vi "pharmaBot_v0.019.vi"() -> ()   [LabVIEW 2015] (continued)
        n1090 = property on="Accept Button" class="Bool (strict)"("DisabledEnum"=T56."Enabled" ("Disabled")) -> ()  [unwired: 2 in, 2 out]
      }
      event "Cancel Calibration Button", "Redo Calibration Button": Mouse Up {
        n1091 = event-data() -> ()  [unwired: 1 in, 8 out]
        n1092 = local write "Calibration Protocol"(T7."Init" ("Calibration Protocol")) -> ()
        n1093 = property on="Accept Button" class="Bool (strict)"("DisabledEnum"=T56."Enabled" ("Disabled")) -> ()  [unwired: 2 in, 2 out]
        n1094 = local write "Stage zeroed?"(FALSE ("Stage zeroed")) -> ()
        n1095 = invoke on="Manip 3 Calibrated" class="Bool (strict)" method="Reinit To Default"() -> ()  [unwired: 3 in, 3 out]
        n1096 = invoke on="Manip 2 Calibrated" class="Bool (strict)" method="Reinit To Default"() -> ()  [unwired: 3 in, 3 out]
        n1097 = invoke on="Manip 1 Calibrated" class="Bool (strict)" method="Reinit To Default"() -> ()  [unwired: 3 in, 3 out]
        n1098 = invoke on="Manip 4 Calibrated" class="Bool (strict)" method="Reinit To Default"() -> ()  [unwired: 3 in, 3 out]
        n1099 = invoke on="Stage zeroed?" class="Bool (strict)" method="Reinit To Default"() -> ()  [unwired: 3 in, 3 out]
      }
      event "wash bath location", "set safe space", "location above baths", "cleaning bath location", "Zero Pipette 1": Mouse Up {
        n1100 = event-data() -> ()  [unwired: 1 in, 8 out]
        n1101 = property on="Accept Button" class="Bool (strict)"("DisabledEnum"=T56."Enabled" ("Disabled")) -> ()  [unwired: 2 in, 2 out]
      }
      event "Pipette is in Focus": Value Change {
        n1102 = event-data() -> ("NewVal"=w1408:bool)  [unwired: 1 in, 5 out]
        n1103 = case shown="True" w1408 {
          frame False {
          }
          frame True {
            n1104 = local read "Current Manipulator Position"() -> (→"Current Manip Focus Coords.":i32[])
            n1105 = local write "Pipette is in Focus?"(TRUE ("Pipette is in Focus?")) -> ()
          }
        }
      }
      event "Move Stage and Pipette Down": Value Change {
        n1106 = event-data() -> ("NewVal"=w1413:bool)  [unwired: 1 in, 5 out]
        n1107 = case shown="True" w1413 {
          tunnel: w1412 -> [_ w1427]
          tunnel: w1411 -> [_ w1426]
          frame False {
          }
          frame True {
            # "manip <z>"
            # "Shift stage by deltaZ"
            # "manip position <x,y>"
            # "calculate deltaZ, reset min on slider"
            # "stage position <x,y>"
            n1108 = local read "current stage pos (steps)"() -> (w1437:i32[])
            n1109 = local read "Next Stage and Pipette Z Location"() -> (w1439:dbl)
            n1110 = local read "Current Manipulator Position"() -> (w1433:i32[])
            n1111 = Index Array(array=w1437, index=2) -> (element=w1434:i32)
            n1112 = Array Subset(array=w1437, length=2) -> (w1430:i32[])  [unwired: 1 in]
            n1113 = Array Subset(array=w1433, length=2) -> (w1429:i32[])  [unwired: 1 in]
            n1114 = Round To Nearest(number=w1439) -> (nearest integer value=w1428:dbl)
            n1115 = flat-sequence {
              tunnel: w1427 -> [w1445]
              tunnel: w1426 -> [w1440]
              tunnel: w1425 -> [w1443]
              tunnel: [w1441] -> w1424
              tunnel: [w1440] -> w1423
              tunnel: w1424 -> [_]
              tunnel: w1423 -> [w1452]
              tunnel: w1422 -> [w1448]
              tunnel: [w1446] -> _
              frame #0 {
                # "move the pipette..."
                n1116 = local read "Calibrate:"() -> (w1444:T8)
                n1117 = call "move manipulator abs xyz.vi"("blocking?"=TRUE, "which manipulator"=w1444, "transform cluster + actuator"=w1440, "positions"=w1445, "location (steps)"=w1443) -> ("error out"=w1441:errorcluster)  [unwired: 6 in]
              }
              frame #1 {
                # "then the stage..."
                n1118 = Unbundle By Name(w1452) -> ("s"=w1451:refnum<vi>)
                n1119 = property class="Clust (strict)"(reference=w1451) -> ("Value"=w1450:T25)  [unwired: 1 in, 2 out]
                n1120 = Unbundle By Name(w1450) -> ("actuator"=w1449:T26)
                n1121 = call "moveTo_abs_XYZ.vi"("blocking?"=TRUE, "XYZ location (steps)"=w1448, "Actuator cluster in"=w1449) -> ("error out"=w1446:errorcluster)  [unwired: 7 in, 1 out]
              }
            }
            n1122 = Subtract(x=w1434, y=w1428) -> (x-y=w1418:dbl)
            n1123 = Index Array(array=w1433, index=2) -> (element=w1432:i32)
            n1124 = Divide(x=w1418, y=7.53) -> (x/y=w1416:dbl)
            n1125 = Subtract(x=w1432, y=w1416) -> (x-y=w1415:dbl)
            n1126 = Subtract(x=w1434, y=w1418) -> (x-y=w1421:dbl)
            n1127 = Negate(x=w1415) -> (-x=w1414:dbl)
            n1128 = Multiply(x=w1421, y=1.0) -> (x*y=w1419:dbl)
            n1129 = Build Array (concatenate)(w1429, w1414) -> (w1425:dbl[])
            "next manip position" <- w1425
            n1130 = Build Array (concatenate)(w1430, w1419) -> (w1422:dbl[])
            "next stage position" <- w1422
          }
        }
      }
      event "Stage Shift (steps)": Value Change {
        n1131 = event-data() -> ("NewVal"=w1453:dbl)  [unwired: 1 in, 5 out]
        n1132 = property on="Next Stage and Pipette Z Location" class="Slide (strict)"("Scale.Maximum"=w1453) -> ()  [unwired: 2 in, 2 out]
      }
      event "Accept Button": Mouse Up {
        n1133 = event-data() -> ()  [unwired: 1 in, 8 out]
        n1134 = property on="Accept Button" class="Bool (strict)"("DisabledEnum"=T56."Disabled and Grayed Out" ("Disabled")) -> ()  [unwired: 2 in, 2 out]
      }
      event "Seek Backwards Calibration Button": Mouse Up {
        n1135 = event-data() -> ()  [unwired: 1 in, 8 out]
        n1136 = local read "Calibration Protocol"() -> (w1457:T7)
        n1137 = Decrement(x=w1457) -> (x-1=w1456:T7)
        n1138 = local write "Calibration Protocol"(w1456) -> ()
        n1139 = property on="Accept Button" class="Bool (strict)"("DisabledEnum"=T56."Disabled and Grayed Out" ("Disabled")) -> ()  [unwired: 2 in, 2 out]
      }
    }
  }
  n1140 = Merge Errors(w395, w396) -> (w397:errorcluster)
  n1141 = case shown="True" w253 {
    tunnel: w467 -> [_ w1466]
    tunnel: w245 -> [_ w1465]
    tunnel: w520 -> [_ w1464]
    tunnel: w518 -> [_ w1463]
    tunnel: w249 -> [_ w1462]
    tunnel: T8."manipulator 2" ("which manipulator") -> [_ w1461]
    tunnel: w281 -> [_ w1460]
    tunnel: w278 -> [_ _]
    frame False {
    }
    frame True {
      n1142 = Current VI's Path() -> (path=w1459:path)
      n1143 = control-ref of="allMainVIcontrols"() -> (w1458:refnum<vi>)
      n1144 = call "multipatch_states_V0.030_dualWCedits.vi"("common cluster"=w1465, "images"=w1466, "allMainVIcontrols"=w1458, "which manipulator"=w1461, "individual controls in"=w1462, "state in"=w1463, "cam size"=w1460, "time in"=w1464, "mainVIpath"=w1459) -> ()  [unwired: 6 in, 1 out]
    }
  }
  n1145 = local write "pipette 2 template"(w267) -> ()
  n1146 = local read "Adjust exposure (ms)"() -> (w275:dbl)
  n1147 = Not(x=w703) -> (.not. x?=→"initialized":bool)
  n1148 = case shown="True" w251 {
    tunnel: w471 -> [_ w1475]
    tunnel: w245 -> [_ w1474]
    tunnel: w520 -> [_ w1473]
    tunnel: w518 -> [_ w1472]
    tunnel: w246 -> [_ w1471]
    tunnel: T8."manipulator 1" ("which manipulator") -> [_ w1470]
    tunnel: w281 -> [_ w1469]
    tunnel: w278 -> [_ _]
    frame False {
    }
    frame True {
      n1149 = Current VI's Path() -> (path=w1468:path)
      n1150 = control-ref of="allMainVIcontrols"() -> (w1467:refnum<vi>)
      n1151 = call "multipatch_states_V0.030_dualWCedits.vi"("common cluster"=w1474, "images"=w1475, "allMainVIcontrols"=w1467, "which manipulator"=w1470, "individual controls in"=w1471, "state in"=w1472, "cam size"=w1469, "time in"=w1473, "mainVIpath"=w1468) -> ()  [unwired: 6 in, 1 out]
    }
  }
  n1152 = while {
    tunnel: w378 -> [w1502]
    tunnel: w336 -> [w1501]
    tunnel: w338 -> [w1495]
    stop <- w1507 stop-if-true
    n1153 = local read "measured manip 1 zero (steps)"() -> (w1497:i32[])
    n1154 = local read "measured stage zero (steps)"() -> (w1496:i32[])
    n1155 = call "get_XYZ.vi"("Actuator cluster in"=w1495) -> ("X pos (steps)"=w1494:i32, "Y pos (steps)"=w1493:i32, "Z pos (steps)"=w1492:i32)  [unwired: 10 in, 2 out]
    n1156 = call "get_XYZ.vi"("Actuator cluster in"=w1502) -> ("X pos (steps)"=w1506:i32, "Y pos (steps)"=w1505:i32, "Z pos (steps)"=w1500:i32)  [unwired: 10 in, 2 out]
    n1157 = call "get_XYZ.vi"("Actuator cluster in"=w1501) -> ("X pos (steps)"=w1504:i32, "Y pos (steps)"=w1503:i32, "Z pos (steps)"=w1499:i32)  [unwired: 10 in, 2 out]
    n1158 = Build Array(w1506, w1505, w1500) -> (w1498:i32[])
    n1159 = Build Array(w1504, w1503, w1499) -> (w1486:i32[])
    n1160 = Build Array(w1494, w1493, w1492) -> (w1491:i32[])
    n1161 = Subtract(x=w1498, y=w1497) -> (x-y=w1477:i32[])
    n1162 = Subtract(x=w1486, y=w1496) -> (x-y=w1478:i32[])
    n1163 = local write "current manip 2 pos (steps)"(w1491) -> ()
    n1164 = local write "measured stage difference (steps)"(w1478) -> ()
    n1165 = local write "current manip 1 pos (steps)"(w1498) -> ()
    n1166 = local write "current stage pos (steps)"(w1486) -> ()
    n1167 = call-poly <vilib>:"nrm2 - Vector 2-Norm.vi"("x"=w1477) -> ("dnrm2"=w1476:dbl)  [unwired: 9 in, 1 out]
    n1168 = call-poly <vilib>:"nrm2 - Vector 2-Norm.vi"("x"=w1478) -> ("dnrm2"=w1479:dbl)  [unwired: 9 in, 1 out]
    n1169 = local write "stage distance (steps)"(w1479) -> ()
    n1170 = local write "measured manip 1 difference (steps)"(w1477) -> ()
    n1171 = local read "stop always"() -> (w1507:bool)
    n1172 = local write "manip distance (steps)"(w1476) -> ()
    n1173 = Index Array(array=w1486, index=2) -> (element=w1484:i32)
    n1174 = Array Subset(array=w1486, length=2) -> (w1483:i32[])  [unwired: 1 in]
    n1175 = Wait (ms)(milliseconds to wait=u32 100) -> ()  [unwired: 1 out]
    n1176 = Divide(x=w1484, y=-75.3) -> (x/y=w1488:dbl)
    n1177 = Divide(x=w1483, y=10 ("Z pos (steps)")) -> (x/y=w1481:dbl[])
    n1178 = Insert Into Array(array=w1481, index=2, new element=w1488) -> (w1480:dbl[])
    n1179 = local write "current stage pos [um]"(w1480) -> ()
  }
  n1180 = And(x=w251, y=w253) -> (x .and. y?=w411:bool)
  n1181 = Bundle By Name(cluster=T38 {"camera type"=enum."optiMOS", "cam handle"=16842752, "data handle"=0, "cam size"=[]} ("cam info in"), "camera type"=w277) -> (w662:T38)
  n1182 = call "init_cam_topLvl_v02.vi"("exposure (ms)"=w275, "orig image"=w276, "cam info in"=w662) -> ("error out"=w280:errorcluster, "cam info out"=w273:T38)  [unwired: 7 in]
  n1183 = Unbundle By Name(w273) -> ("cam size"=w328:i32[])
  n1184 = call "IMAQ Create"("Border Size"=0, "Image Name"="correctionMask", "Image Type"=w332, "error in (no error)"=w333) -> ("New Image"=w329:T10, "error out"=w330:errorcluster)  [unwired: 1 in]
  n1185 = call <vilib>:"Set Plots.vi"("3D graph"=w271, "# of plots(1)"=7) -> ("3D graph out"=w666:refnum<k7>, "error out"=w665:errorcluster)  [unwired: 12 in]
  n1186 = local write "Select cells based on proximity (multi patch)"(w411) -> ()
  n1187 = local read "cell diameter (px)"() -> (w274:i32)
  n1188 = local write "cam info out"(w273) -> ()
  n1189 = Index Array(array=w328) -> (element #1=w327:i32, element #2=w326:i32)  [unwired: 2 in]
  n1190 = call "condition3dplot_v02.vi"("error in"=w665, "3d graph"=w666) -> ("3d graph out"=w664:refnum<k7>)  [unwired: 8 in, 1 out]
  n1191 = property class="CWGraph3D"(reference=w271) -> ("Axes"=w635:refnum<k7>)  [unwired: 1 in, 2 out]
  n1192 = call "IMAQ SetImageSize"("error in (no error)"=w330, "Y Resolution"=w326, "X Resolution"=w327, "Image"=w329) -> ("error out"=w325:errorcluster, "Image Out"=w324:T10)  [unwired: 1 in]
  n1193 = Select(t=scope_motion."slow_dualPatch" ("motion"), s=w411, f=scope_motion."slow_dualPatch" ("motion")) -> (s? t:f=w248:T19)
  n1194 = flat-sequence {
    tunnel: [w1513] -> w637
    tunnel: [w1512] -> w636
    tunnel: w273 -> [w1511]
    tunnel: w280 -> [w1510]
    tunnel: [w1510] -> w279
    frame #0 {
      n1195 = Unbundle By Name(w1511) -> ("cam size"=w1509:i32[])
      n1196 = Index Array(array=w1509) -> (element #1=w1513:i32, element #2=w1512:i32)  [unwired: 2 in]
      n1197 = local write "cam size"(w1509) -> ()
      n1198 = property on="camera" class="XYGraph (strict)"("XScale.Maximum"=w1513, "YScale.Maximum"=w1512) -> ()  [unwired: 2 in, 2 out]
    }
  }
  n1199 = call "init_camCorrection.vi"("error in"=w325, "orig image"=w324, "cam info in"=w273) -> ("error out"=w282:errorcluster, "orig image out"=w323:T10)  [unwired: 7 in]
  n1200 = local write "pipette motion"(w248) -> ()
  n1201 = To Variant(anything=1) -> (Variant=w644:variant)
  n1202 = To Variant(anything=2) -> (Variant=w642:variant)
  n1203 = local read "Valve2 Connected"() -> (w283:bool)
  n1204 = invoke class="CWAxes3D" method="Item"(reference=w635, "Item"=w642) -> ("Item"=w640:refnum<k7>)  [unwired: 2 in, 3 out]
  n1205 = invoke class="CWAxes3D" method="Item"(reference=w635, "Item"=w644) -> ("Item"=w643:refnum<k7>)  [unwired: 2 in, 3 out]
  n1206 = local read "P1 state"() -> (w356:T11)
  n1207 = while {
    tunnel: w276 -> [w1547]
    tunnel: [w1521] -> w681
    tunnel: [w1523] -> w680
    tunnel: [w1554] -> w677
    tunnel: [w1553] -> w676
    tunnel: w274 -> [w1555]
    tunnel: w366 -> [w1520]
    tunnel: w273 -> [w1548]
    tunnel: w280 -> [w1546]
    tunnel: [w1525] -> w660
    shift-right: [w1516] -> _
    shift-left: sgl[] [] ("Distances") -> [w1537]
    tunnel: w275 -> [w1529]
    tunnel: w282 -> [_]
    tunnel: w323 -> [w1519]
    stop <- w1559 stop-if-true
    w1541 = i32[] [2] items=["No Event"=0, "Click Event"=1, "Draw Event"=2, "Size Event"=4, "Scroll Event"=5, "Double Click Event"=8] ("Which Events")
    # "draws circle where it found tip\nduring auto pipette calibration"
    # "if cell tracker is ON\nplot outline, centroid, pipette position"
    n1208 = local read "Vision Fix"() -> (w1526:bool)
    n1209 = call "grab_image_topLvl_v02.vi"("error in"=w1546, "orig image"=w1547, "cam info in"=w1548) -> ("error out"=w1522:errorcluster, "orig image out"=w1524:T10, "cam info out"=w1525:T38)  [unwired: 6 in]
    n1210 = Multiply(x=w1529, y=1.1) -> (x*y=w1527:dbl)
    n1211 = case shown="True" w1526 {
      tunnel: w1524 -> [w1561 w1563]
      tunnel: [w1561 w1567] -> w1523
      tunnel: w1522 -> [w1560 w1565]
      tunnel: [w1560 w1564] -> w1521
      tunnel: w1520 -> [_ w1566]
      tunnel: w1519 -> [_ w1562]
      frame False {
      }
      frame True {
        n1212 = call "IMAQ Multiply"("Image Src A"=w1563, "Image Dst"=w1566, "Image Src B"=w1562, "error in (no error)"=w1565) -> ("Image Dst Out"=w1567:T10, "error out"=w1564:errorcluster)  [unwired: 3 in]
      }
    }
    n1213 = Wait (ms)(milliseconds to wait=w1527) -> ()  [unwired: 1 out]
    n1214 = call "IMAQ Copy"("error in (no error)"=w1521, "Image Dst"=w1520, "Image Src"=w1523) -> ("error out"=w1545:errorcluster, "Image Dst Out"=w1544:T10)  [unwired: 3 in]
    n1215 = local read "crosshair?"() -> (w1517:bool)
    n1216 = case shown="True" w1517 {
      tunnel: [w1608 w1612] -> w1557
      tunnel: [w1607 w1611] -> w1556
      tunnel: w1544 -> [w1608 w1610]
      tunnel: w1545 -> [w1607 w1609]
      frame False {
      }
      frame True {
        n1217 = call "overlayCrosshairs.vi"("error in"=w1609, "Image in"=w1610) -> ("error out"=w1611:errorcluster, "Image out"=w1612:T10)  [unwired: 8 in]
      }
    }
    n1218 = local read "current cell locations (px)"() -> (w1558:dbl[][])
    n1219 = invoke on="Slice view" class="ImageControl" method="Get Last Event"("Which Events"=w1541) -> ("Tool"=w1536:i32, "Coordinates"=w1540:i32[])  [unwired: 7 in, 6 out]
    n1220 = call "drawCells.vi"("error in"=w1556, "diameter (px)"=w1555, "current cell locations (px)"=w1558, "Image in"=w1557) -> ("error out"=w1539:errorcluster, "Image out"=w1542:T10)  [unwired: 6 in]
    n1221 = case shown="3" w1536 {
      tunnel: w1540 -> [_ w1574]
      tunnel: w1539 -> [w1569 w1573]
      tunnel: [w1569 w1572] -> w1538
      tunnel: [w1568 w1570] -> w1516
      tunnel: w1537 -> [w1568 _]
      frame 0, Default {
      }
      frame 3 {
        w1571 = cluster{"X":sgl, "Y":sgl} {"X"=0.0, "Y"=0.0}
        # "Line tool"
        # "IMAQ Point Distances"
        n1222 = Index Array(array=w1574, index #1=0 ("index"), index #2=1 ("index"), index #3=2 ("index"), index #4=3 ("index")) -> (element #1=w1579:i32, element #2=w1580:i32, element #3=w1581:i32, element #4=w1582:i32)
        n1223 = Bundle(cluster=w1571, "X"=w1581, "Y"=w1582) -> (w1583:cluster{"X":sgl, "Y":sgl})
        n1224 = Bundle(cluster=w1571, "X"=w1579, "Y"=w1580) -> (w1584:cluster{"X":sgl, "Y":sgl})
        n1225 = Build Array(w1583, w1584) -> (w1585:cluster{"X":sgl, "Y":sgl}[])
        n1226 = call "IMAQ Point Distances"("Points"=w1585, "error in (no error)"=w1573) -> ("Distances"=w1570:sgl[], "error out"=w1572:errorcluster)  [unwired: 3 in]
      }
    }
    n1227 = local read "tracking"() -> (w1543:bool)
    n1228 = case shown="False" w1543 {
      tunnel: w1542 -> [w1587 w1605]
      tunnel: w1538 -> [w1586 w1604]
      tunnel: [w1586 w1588] -> w1534
      tunnel: [w1587 w1589] -> w1535
      frame False {
      }
      frame True {
        n1229 = local read "cell mask ROI"() -> (w1606:T28)
        n1230 = local read "centroid_px"() -> (w1598:dbl[])
        n1231 = call "IMAQ Overlay ROI"("error in (no error)"=w1604, "ROI Descriptor"=w1606, "Image"=w1605) -> ("error out"=w1599:errorcluster, "Image Out"=w1600:T10)  [unwired: 7 in]
        n1232 = To Long Integer(number=w1598) -> (32bit integer=w1597:i32[])
        n1233 = call "boundingBoxCoords.vi"("side length (px)"=20, "center (x,y)"=w1597) -> ("bounding box"=w1601:T59)  [unwired: 8 in, 1 out]
        n1234 = local read "pipette_px_onscreen"() -> (w1592:dbl[])
        n1235 = call "IMAQ Overlay Oval"("Color"=u32 6618880, "error in (no error)"=w1599, "Bounding Rectangle"=w1601, "Image"=w1600) -> ("error out"=w1590:errorcluster, "Image Out"=w1591:T10)  [unwired: 6 in]
        n1236 = To Long Integer(number=w1592) -> (32bit integer=w1596:i32[])
        n1237 = call "boundingBoxCoords.vi"("side length (px)"=10, "center (x,y)"=w1596) -> ("bounding box"=w1595:T59)  [unwired: 8 in, 1 out]
        n1238 = call "IMAQ Overlay Oval"("Color"=u32 9567230, "error in (no error)"=w1590, "Bounding Rectangle"=w1595, "Image"=w1591) -> ("error out"=w1588:errorcluster, "Image Out"=w1589:T10)  [unwired: 6 in]
      }
    }
    n1239 = local write "Distances"(w1516) -> ()
    n1240 = local read "Range"() -> (w1515:cluster{"Minimum":sgl, "Maximum":sgl})
    n1241 = call "IMAQ MathLookup"("Range"=w1515, "Operator"=T58."Linear", "error in (no error)"=w1534, "Image Src"=w1535) -> ("error out"=w1532:errorcluster, "Image Dst Out"=w1518:T10)  [unwired: 6 in]
    n1242 = call "IMAQ Histograph"("Interval Range"=w1515, "Image"=w1518) -> ("Histogram Graph"=w1514:T21)  [unwired: 6 in, 3 out]
    n1243 = local read "screen tip location (px)"() -> (w1549:i32[])
    n1244 = local write "Waveform Graph"(w1514) -> ()
    n1245 = local write "Slice view"(w1518) -> ()
    n1246 = local read "stop always"() -> (w1559:bool)
    n1247 = call "_Adjust Dynamic_simple.vi"("error in (no error)"=w1532, "Image Src"=w1518) -> ("error out"=w1531:errorcluster, "Image Out"=w1530:T10)  [unwired: 8 in]
    n1248 = call "boundingBoxCoords.vi"("side length (px)"=20, "center (x,y)"=w1549) -> ("bounding box"=w1551:T59)  [unwired: 8 in, 1 out]
    n1249 = call "IMAQ Overlay Oval"("Color"=u32 16711680, "error in (no error)"=w1531, "Bounding Rectangle"=w1551, "Image"=w1530) -> ("error out"=w1553:errorcluster, "Image Out"=w1554:T10)  [unwired: 6 in]
  }
  n1250 = local read "P1 state"() -> (w353:T11)
  n1251 = Not Equal?(x=w353, y=user_message_v6."Setting defaults..." ("P1 state")) -> (x != y?=w357:bool)
  n1252 = Not Equal?(x=w356, y=user_message_v6."Initializing..." ("P1 state")) -> (x != y?=w358:bool)
  n1253 = Or(x=w357, y=w358) -> (x .or. y?=w285:bool)
  n1254 = Select(t=w285, s=w283, f=w283) -> (s? t:f=w284:bool)
  n1255 = control-ref of="Command pressure (mBar) 1"() -> (w670:refnum<vi>)
  n1256 = while {
    tunnel: w270 -> [w1623]
    tunnel: w272 -> [w1622]
    tunnel: w664 -> [w1619]
    tunnel: [w1619] -> w663
    stop <- w1621 stop-if-true
    n1257 = local read "park plane z (px)"() -> (w1618:dbl)
    n1258 = local read "cells (image px)"() -> (w1620:dbl[][])
    n1259 = call "cam5_3dTest.vi"("park plane z (px)"=w1618, "3d graph"=w1619, "transform cluster + actuator"=w1622, "positions"=w1623, "cells (image px locations)"=w1620) -> ("current stage location (px)"=w1613:dbl[], "current pipette locations (px)"=w1614:dbl[][], "current cell locations (px)"=w1615:dbl[][], "currentState out"=w1616:T33, "current park plane z (px)"=w1617:dbl)  [unwired: 2 in]
    n1260 = local write "current park plane z (px)"(w1617) -> ()
    n1261 = local write "camera"(w1616) -> ()
    n1262 = local write "current cell locations (px)"(w1615) -> ()
    n1263 = local write "current pipette locations (px)"(w1614) -> ()
    n1264 = local write "current stage location (px)"(w1613) -> ()
    n1265 = local read "stop always"() -> (w1621:bool)
    n1266 = Wait (ms)(milliseconds to wait=u32 100) -> ()  [unwired: 1 out]
  }
  n1267 = call "Time Delay2"("Delay Time (s)"=2.0) -> ("error out"=w701:errorcluster)  [unwired: 10 in]
  n1268 = To Variant(anything=w636) -> (Variant=w638:variant)
  n1269 = To Variant(anything=w637) -> (Variant=w639:variant)
  n1270 = property class="CWAxis3D"(reference=w640, "Maximum"=w638) -> ()  [unwired: 1 in, 2 out]
  n1271 = property class="CWAxis3D"(reference=w643, "Maximum"=w639) -> ()  [unwired: 1 in, 2 out]
  n1272 = local read "demo daq?"() -> (w247:bool)
  n1273 = control-ref of="Command pressure (mBar) 2"() -> (w482:refnum<vi>)
  n1274 = while {
    tunnel: w696 -> [w1649]
    tunnel: w266 -> [w1648]
    tunnel: w627 -> [w1647]
    tunnel: w270 -> [w1646]
    tunnel: w272 -> [w1645]
    tunnel: w672 -> [w1644]
    tunnel: w322 -> [w1643]
    tunnel: w670 -> [w1642]
    tunnel: w265 -> [w1641]
    tunnel: w621 -> [w1640]
    tunnel: w482 -> [w1639]
    tunnel: w267 -> [w1638]
    tunnel: w464 -> [w1637]
    tunnel: w269 -> [w1636]
    tunnel: w456 -> [w1635]
    tunnel: w432 -> [w1634]
    tunnel: w431 -> [w1633]
    tunnel: w394 -> [w1632]
    tunnel: w398 -> [w1631]
    tunnel: [w1630] -> w401
    tunnel: [w1629] -> w400
    tunnel: w366 -> [w1628]
    tunnel: w337 -> [w1627]
    tunnel: w246 -> [w1626]
    tunnel: w245 -> [w1625]
    stop <- w1650 stop-if-true
    n1275 = event shown="[29] \"MZ Dn\", \"MZ Up\", \"MX Up\", \"MX Dn\", \"MY Dn\", \"MY Up\", \"SZ Dn\", \"SZ Up\", \"SX Up\", \"SX Dn\", \"SY Dn\", \"SY Up\": Value Change" {
      selector: _ -> [_ _ _ _ _ _ _ _ _ _ _ _ _ _ _ _ _ _ _ _ _ _ _ _ _ _ _ _ _ _ _ _ _ _ _ _ _ _ _ _ _]
      dyn-events: _ -> [_ _ _ _ _ _ _ _ _ _ _ _ _ _ _ _ _ _ _ _ _ _ _ _ _ _ _ _ _ _ _ _ _ _ _ _ _ _ _ _ _]
      timeout: _ -> [_ _ _ _ _ _ _ _ _ _ _ _ _ _ _ _ _ _ _ _ _ _ _ _ _ _ _ _ _ _ _ _ _ _ _ _ _ _ _ _ _]
      tunnel: [w1653 FALSE ("stop events") TRUE ("stop events") FALSE ("stop events") FALSE ("stop events") TRUE ("stop events") FALSE ("stop events") FALSE ("stop events") FALSE ("stop events") FALSE ("stop events") _ FALSE ("stop events") FALSE ("stop events") FALSE ("stop events") FALSE ("stop events") FALSE ("stop events") FALSE ("stop events") FALSE ("stop events") FALSE ("stop events") FALSE ("stop events") FALSE ("stop events") FALSE ("stop events") FALSE ("stop events") FALSE ("stop events") FALSE ("stop events") FALSE ("stop events") FALSE ("stop events") FALSE ("stop events") FALSE ("stop events") FALSE ("stop events") FALSE ("stop events") FALSE ("stop events") FALSE ("stop events") FALSE ("stop events") _ _ FALSE ("stop events") FALSE ("stop events") FALSE ("stop events") FALSE ("stop events") FALSE ("stop events")] -> w1650
      tunnel: w1649 -> [_ _ _ _ _ _ _ _ _ _ _ _ _ _ _ _ _ _ _ _ _ _ w2190 w2219 _ _ _ _ _ _ _ _ w2703 _ _ _ _ _ _ _ _]
      tunnel: w1648 -> [_ _ _ _ _ _ w1723 _ _ _ _ _ _ _ _ _ _ _ _ _ _ _ _ _ _ _ _ _ _ _ _ _ _ _ _ _ _ _ _ _ _]
      tunnel: w1647 -> [_ _ _ _ _ _ w1727 _ _ _ _ _ _ _ _ _ _ _ _ _ _ _ _ _ _ _ _ _ _ _ _ _ _ _ _ _ _ _ _ _ _]
      tunnel: w1646 -> [_ _ w1661 _ _ w1695 w1726 _ _ w1915 _ _ _ _ _ _ _ _ _ _ _ w2170 w2192 w2221 w2246 w2275 _ w2341 w2380 w2416 w2642 w2670 _ _ _ _ _ _ _ _ w2866]
      tunnel: w1645 -> [_ _ w1662 _ _ w1696 w1725 w1895 _ w1914 _ _ _ _ _ w1986 w2022 w2092 w2112 w2132 w2147 w2169 w2193 w2222 w2249 w2278 w2308 w2342 w2381 w2417 w2643 w2669 _ _ _ _ _ _ _ _ w2865]
      tunnel: w1644 -> [_ _ _ _ _ _ _ _ _ _ _ _ _ w1951 _ _ _ _ _ _ _ _ _ _ _ _ _ _ _ _ _ _ _ _ _ _ _ _ _ _ _]
      tunnel: w1643 -> [_ _ w1664 w1687 w1691 w1698 _ _ _ _ _ _ _ _ _ _ _ _ _ _ _ _ _ _ _ _ _ _ _ _ _ _ _ _ _ _ _ _ _ _ _]
      tunnel: w1642 -> [_ _ w1663 w1686 _ w1697 _ _ _ _ _ _ _ _ _ _ _ _ _ _ _ _ _ _ _ _ _ _ _ _ _ _ _ _ _ _ _ _ _ _ _]
      tunnel: w1641 -> [_ _ _ _ _ _ w1724 _ _ _ _ _ _ _ _ _ _ _ _ _ _ _ _ _ _ _ _ _ _ _ _ _ _ _ _ _ _ _ _ _ _]
      tunnel: w1640 -> [_ _ _ _ _ _ w1722 _ _ _ _ _ _ _ _ _ _ _ _ _ _ _ _ _ _ _ _ _ _ _ _ _ _ _ _ _ _ _ _ _ _]
      tunnel: w1639 -> [_ _ _ _ w1690 w1694 _ _ _ _ _ _ _ _ _ _ _ _ _ _ _ _ _ _ _ _ _ _ _ _ _ _ _ _ _ _ _ _ _ _ _]
      tunnel: w1638 -> [_ _ _ _ _ _ w1721 _ _ _ _ _ _ _ _ _ _ _ _ _ _ _ _ _ _ _ _ _ _ _ _ _ _ _ _ _ _ _ _ _ _]
      tunnel: w1637 -> [_ _ _ _ _ _ w1720 _ _ _ _ _ _ _ _ _ _ _ _ _ _ _ _ _ _ _ _ _ _ _ _ _ _ _ _ _ _ _ _ _ _]
      tunnel: w1636 -> [_ _ _ _ _ _ w1719 _ _ _ _ _ _ _ _ _ _ _ _ _ _ _ _ _ _ _ _ _ _ _ _ _ _ _ _ _ _ _ _ _ _]
      tunnel: w1635 -> [_ _ _ _ _ _ w1718 _ _ _ _ _ _ _ _ _ _ _ _ _ _ _ _ _ _ _ _ _ _ _ _ _ _ _ _ _ _ _ _ _ _]
      tunnel: w1634 -> [_ _ _ _ _ _ w1716 _ _ _ _ _ _ _ _ _ _ _ _ _ _ _ _ _ _ _ _ _ _ _ _ _ _ _ _ _ _ _ _ _ _]
      tunnel: w1633 -> [_ _ _ _ _ _ w1715 _ _ _ _ _ _ _ _ _ _ _ _ _ _ _ _ _ _ _ _ _ _ _ _ _ _ _ _ _ _ _ _ _ _]
      tunnel: w1632 -> [w1655 _ _ _ _ _ _ _ _ _ _ _ _ _ _ _ _ _ _ _ _ _ _ _ _ _ _ _ _ _ _ _ _ _ _ _ _ _ _ _ _]
      tunnel: w1631 -> [w1654 w1658 _ _ _ _ _ _ _ _ _ _ _ _ _ _ _ _ _ _ _ _ _ _ _ _ _ _ _ _ _ _ _ _ _ _ _ _ _ _ _]
      tunnel: [w1652 _ _ _ _ _ _ _ _ _ _ _ _ _ _ _ _ _ _ _ _ _ _ _ _ _ _ _ _ _ _ _ _ _ _ _ _ _ _ _ _] -> w1630
      tunnel: [w1651 w1658 _ _ _ _ _ _ _ _ _ _ _ _ _ _ _ _ _ _ _ _ _ _ _ _ _ _ _ _ _ _ _ _ _ _ _ _ _ _ _] -> w1629
      tunnel: w1628 -> [_ _ _ _ _ _ w1714 w1896 _ w1913 _ _ _ _ _ _ w2021 _ _ _ _ _ _ _ _ _ _ _ _ _ _ _ _ _ _ _ _ _ _ _ _]
      tunnel: w1627 -> [_ _ _ _ _ _ _ _ _ _ _ _ _ _ _ _ _ _ _ _ _ _ w2191 w2220 w2248 w2277 _ _ _ _ _ _ _ _ _ _ _ _ _ _ _]
      tunnel: w1626 -> [_ _ _ _ _ _ _ _ _ _ _ _ _ _ _ _ _ _ _ _ _ _ w2189 w2218 w2247 w2276 _ _ _ _ _ _ _ _ _ _ _ _ _ _ _]
      tunnel: w1625 -> [_ _ _ _ _ _ _ _ _ _ _ _ _ _ _ _ _ _ _ _ _ _ w2188 w2217 _ _ _ _ _ _ _ _ _ _ _ _ _ _ _ _ _]
      event "stop": Value Change {
        w1653 = TRUE ("stop events")
        n1276 = event-data() -> ()  [unwired: 1 in, 5 out]
        n1277 = Send Notification(notification=w1653, notifier=w1655, error in (no error)=w1654) -> (notifier out=w1652:refnum<notifier>, error out=w1651:errorcluster)
        "stop always" <- TRUE ("stop always")
      }
      event Timeout {
        n1278 = event-data() -> ()  [unwired: 1 in, 3 out]
        n1279 = Wait (ms)(milliseconds to wait=u32 50) -> ()  [unwired: 1 out]
      }
      event "pipette 1 broken - abort!": Value Change {
        n1280 = event-data() -> ("NewVal"=w1665:bool)  [unwired: 1 in, 5 out]
        n1281 = case shown="True" w1665 {
          tunnel: w1664 -> [_ w1681]
          tunnel: w1663 -> [_ w1680]
          tunnel: w1662 -> [_ w1670]
          tunnel: w1661 -> [_ w1676]
          frame False {
          }
          frame True {
            w1675 = T8."manipulator 1" ("which manipulator")
            n1282 = Unbundle By Name(w1670) -> ("manip 1"=w1669:refnum<vi>)
            n1283 = property class="Clust (strict)"(reference=w1669) -> (error out=w1668:errorcluster, "Value"=w1667:T25)  [unwired: 1 in, 1 out]
            n1284 = call "switchPressure_topLvl.vi"("which manipulator"=w1675, "Slide Refnum"=w1680, "error in"=w1668, "pressure setting"=arduino_pressure_setting."Atmospheric Pressure", "Pressure box control in"=w1681) -> ("error out"=w1671:errorcluster)  [unwired: 5 in, 1 out]
            n1285 = Unbundle By Name(w1667) -> ("actuator.Actuator COM"=w1672:refnum<visa-resource-name>)
            n1286 = call "sc_adjustMotion.vi"("error in (no error)"=w1671, "motion"=scope_motion."fast", "VISA handle"=w1672) -> ("error out"=w1666:errorcluster)  [unwired: 7 in, 1 out]
            n1287 = Unbundle By Name(w1667) -> ("safe space (steps)"=w1678:i32[])
            n1288 = call "move manipulator abs xyz.vi"("blocking?"=TRUE, "which manipulator"=w1675, "error in (no error)"=w1666, "transform cluster + actuator"=w1670, "positions"=w1676, "location (steps)"=w1678) -> ("error out"=w1677:errorcluster)  [unwired: 5 in]
            n1289 = flat-sequence {
              tunnel: w1677 -> [_]
              frame #0 {
                n1290 = Stop(stop? (T)=TRUE) -> ()
              }
            }
          }
        }
      }
      event "Command pressure (mBar) 1": Value Change {
        n1291 = event-data() -> ("NewVal"=w1684:dbl)  [unwired: 1 in, 5 out]
        n1292 = call "setPressure_topLvl.vi"("which manipulator"=T8."manipulator 1", "Slide Refnum"=w1686, "set pressure (mBar)"=w1684, "Pressure box control in"=w1687) -> ()  [unwired: 6 in, 2 out]
      }
      event "Command pressure (mBar) 2": Value Change {
        n1293 = event-data() -> ("NewVal"=w1692:dbl)  [unwired: 1 in, 5 out]
        n1294 = call "setPressure_topLvl.vi"("which manipulator"=T8."manipulator 2", "Slide Refnum"=w1690, "set pressure (mBar)"=w1692, "Pressure box control in"=w1691) -> ()  [unwired: 6 in, 2 out]
      }
      event "pipette 2 broken - abort!": Value Change {
        n1295 = event-data() -> ("NewVal"=w1699:bool)  [unwired: 1 in, 5 out]
        n1296 = case shown="True" w1699 {
          tunnel: w1698 -> [_ w1710]
          tunnel: w1697 -> [_ _]
          tunnel: w1696 -> [_ w1703]
          tunnel: w1695 -> [_ w1704]
          tunnel: w1694 -> [_ w1700]
          frame False {
          }
          frame True {
            w1702 = T8."manipulator 2" ("which manipulator")
            n1297 = Unbundle By Name(w1703) -> ("manip 2"=w1706:refnum<vi>)
            n1298 = call "switchPressure_topLvl.vi"("which manipulator"=w1702, "Slide Refnum"=w1700, "pressure setting"=arduino_pressure_setting."Atmospheric Pressure", "Pressure box control in"=w1710) -> ()  [unwired: 6 in, 2 out]
            n1299 = property class="Clust (strict)"(reference=w1706) -> ("Value"=w1708:T25)  [unwired: 1 in, 2 out]
            n1300 = Unbundle By Name(w1708) -> ("safe space (steps)"=w1707:i32[])
            n1301 = call "move manipulator abs xyz.vi"("blocking?"=TRUE, "which manipulator"=w1702, "transform cluster + actuator"=w1703, "positions"=w1704, "location (steps)"=w1707) -> ("error out"=w1705:errorcluster)  [unwired: 6 in]
            n1302 = flat-sequence {
              tunnel: w1705 -> [_]
              frame #0 {
                n1303 = Stop(stop? (T)=TRUE) -> ()
              }
            }
          }
        }
      }
      event "Slice view": Mouse Up {
        # "1 - left\n2 - right\n3 - dial"
        # "pipette 2 template"
        # "pipette 1 template"
        # "pipette 2 mask"
        # "pipette 1 mask"
        n1304 = event-data() -> ("CtlRef"=w1730:refnum<vi>, "Button"=w1713:u16)  [unwired: 1 in]
        n1305 = local read "Calibrate:"() -> (w1717:T8)
        n1306 = local read "which action on cam"() -> (w1729:T6)
        n1307 = property class="ImageControl"(reference=w1730) -> ("Last Mouse Position"=w1728:cluster{"X":i32, "Y":i32})  [unwired: 1 in, 2 out]
        n1308 = case shown="\"Add cell\"" w1729 {
          tunnel: w1728 -> [w1736 w1744 w1863 _]
          tunnel: w1723 -> [_ _ w1852 _]
          tunnel: w1727 -> [_ _ w1853 _]
          tunnel: w1726 -> [w1733 w1741 _ _]
          tunnel: w1725 -> [w1732 w1740 _ _]
          tunnel: w1724 -> [_ _ w1850 _]
          tunnel: w1722 -> [_ _ w1849 _]
          tunnel: w1721 -> [_ _ w1851 _]
          tunnel: w1720 -> [_ _ w1844 _]
          tunnel: w1719 -> [_ _ w1847 _]
          tunnel: w1718 -> [_ _ w1848 _]
          tunnel: w1717 -> [_ _ w1846 _]
          tunnel: w1717 -> [_ _ w1845 _]
          tunnel: w1716 -> [_ _ w1840 _]
          tunnel: w1715 -> [_ _ w1839 _]
          tunnel: w1714 -> [_ w1743 w1826 _]
          tunnel: w1713 -> [_ w1742 _ _]
          frame "Move pipette", Default {
            n1309 = Unbundle By Name(w1736) -> ("X"=w1737:i32, "Y"=w1738:i32)
            n1310 = local read "Calibrate:"() -> (w1731:T8)
            n1311 = Build Array(w1737, w1738) -> (w1739:i32[])
            n1312 = call "camToPipette_abs_3d.vi"("which manipulator"=w1731, "transform cluster + actuator"=w1732, "current positions"=w1733, "abs pixel location"=w1739) -> ("pipette location (steps)"=w1734:dbl[])  [unwired: 7 in]
            n1313 = call "move manipulator abs xy.vi"("blocking?"=TRUE, "which manipulator"=w1731, "transform cluster + actuator"=w1732, "positions"=w1733, "location (steps)"=w1734) -> ()  [unwired: 6 in, 1 out]
          }
          frame "Add cell" {
            n1314 = case shown="1" w1742 {
              tunnel: w1744 -> [_ w1766 w1825]
              tunnel: w1743 -> [_ w1745 _]
              tunnel: w1741 -> [_ _ w1806]
              tunnel: w1740 -> [_ _ w1820]
              frame 0, Default {
              }
              frame 1 {
                w1765 = T47 7 items=["Grayscale (U8)", "Grayscale (I16)", "Grayscale (SGL)", "Complex (CSG)", "RGB (U32)", "HSL (U32)", "RGB (U64)", "Grayscale (U16)"] ("Image Type")
                # "add cell"
                # "get mouse position, make box around it\nthat is the cell. this will be used for pattern matching"
                # "add new cell coordinates\nfirst row is x of all cells\nsecond row is y of all cells"
                n1315 = Cluster To Array(cluster=w1766) -> (array=w1759:i32[])
                n1316 = local read "current stage pos (steps)"() -> (w1776:i32[])
                n1317 = local read "stage->cam"() -> (w1777:T25)
                n1318 = local read "cells (image px)"() -> (w1767:dbl[][])
                n1319 = Index Array(array=w1776) -> (element #1=w1775:i32, element #2=w1774:i32, element #3=w1761:i32)  [unwired: 3 in]
                n1320 = Array Size(array=w1767) -> (size(s)=w1779:i32[])
                n1321 = call "transformCoords_3d.vi"("transform properties"=w1777, "z"=w1761, "y"=w1774, "x"=w1775) -> ("z out"=w1760:dbl, "y out"=w1772:dbl, "x out"=w1773:dbl)  [unwired: 5 in]
                n1322 = Build Array (concatenate)(w1759, 0) -> (w1757:i32[])
                n1323 = Index Array(array=w1779, index=1) -> (element=w1780:i32)
                n1324 = Build Array(w1773, w1772, w1760) -> (w1771:dbl[])
                n1325 = Subtract(x=w1757, y=w1771) -> (x-y=w1770:dbl[])
                n1326 = Build Array(w1770) -> (w1769:dbl[][])
                n1327 = Transpose 2D Array(2D array=w1769) -> (transposed array=w1768:dbl[][])
                n1328 = Insert Into Array(array=w1767, index (col)=w1780, new element=w1768) -> (w1754:dbl[][])  [unwired: 1 in]
                n1329 = Number To Decimal String(number=w1780) -> (decimal integer string=w1764:string)  [unwired: 1 in]
                n1330 = local read "cell images"() -> (w1763:T10[])
                n1331 = call "IMAQ Create"("Image Name"=w1764, "Image Type"=w1765) -> ("New Image"=w1762:T10)  [unwired: 3 in, 1 out]
                n1332 = call "boundingBoxCoords.vi"("side length (px)"="cell image size (px)", "center (x,y)"=w1757) -> ("bounding rectangle"=w1755:i32[])  [unwired: 8 in, 1 out]
                n1333 = call "IMAQ Extract 2"("Optional Rectangle"=w1755, "Image Dst"=w1762, "Image Src"=w1745) -> ("error out"=w1756:errorcluster, "Image Dst Out"=w1753:T10)  [unwired: 7 in]
                n1334 = Decrement(x="cell image size (px)") -> (x-1=w1749:i32)
                n1335 = call "IMAQ GetImageSize"("Image"=w1753) -> ("Y Resolution"=w1751:i32, "X Resolution"=w1750:i32)  [unwired: 3 in, 1 out]
                n1336 = Equal?(x=w1750, y=w1749) -> (x = y?=w1748:bool)
                n1337 = Equal?(x=w1751, y=w1749) -> (x = y?=w1747:bool)
                n1338 = And(x=w1748, y=w1747) -> (x .and. y?=w1746:bool)
                n1339 = case shown="True" w1746 {
                  tunnel: w1763 -> [_ w1792]
                  tunnel: w1756 -> [_ w1790]
                  tunnel: w1753 -> [_ w1789]
                  tunnel: w1754 -> [_ w1782]
                  frame False {
                    n1340 = call "Display Message to User2"() -> ()  [unwired: 10 in, 2 out]
                  }
                  frame True {
                    w1791 = 0 items=["All", "Low Discrepancy Sampling", "Grayscale Value Pyramid", "Gradients Pyramid"] ("Algorithm")
                    # "update unpatched cell indices"
                    n1341 = local write "cells (image px)"(w1782) -> ()
                    n1342 = Array Size(array=w1782) -> (size(s)=w1786:i32[])
                    n1343 = Index Array(array=w1786, index=1) -> (element=w1785:i32)
                    n1344 = call "IMAQ Learn Pattern 5"("Image"=w1789, "Algorithm"=w1791, "error in (no error)"=w1790) -> ("Template Image Out"=w1788:T10)  [unwired: 10 in, 2 out]
                    "saved cell image" <- w1788
                    n1345 = for {
                      N: w1785 -> [_]
                      shift-right: [w1793] -> w1781
                      shift-left: i32[] [] ("manip 1 cell indices 2") -> [w1795]
                      i -> [w1794]
                      n1346 = Build Array (concatenate)(w1795, w1794) -> (w1793:i32[])
                    }
                    n1347 = Insert Into Array(array=w1792, new element=w1788) -> (w1787:T10[])  [unwired: 1 in]
                    n1348 = local write "cell images"(w1787) -> ()
                    n1349 = local write "unpatched cell indices"(w1781) -> ()
                  }
                }
              }
              frame 3 {
                # "move stage"
                n1350 = local read "cam size"() -> (w1818:i32[])
                n1351 = Unbundle By Name(w1806) -> ("current stage pos (steps)"=w1807:refnum<vi>)
                n1352 = Index Array(array=w1818) -> (element #1=w1817:i32, element #2=w1814:i32)  [unwired: 2 in]
                n1353 = Unbundle By Name(w1825) -> ("X"=w1813:i32, "Y"=w1811:i32)
                n1354 = Divide(x=w1817, y=2) -> (x/y=w1812:dbl)
                n1355 = Divide(x=w1814, y=2) -> (x/y=w1810:dbl)
                n1356 = Subtract(x=w1813, y=w1812) -> (x-y=w1809:dbl)
                n1357 = Subtract(x=w1811, y=w1810) -> (x-y=w1808:dbl)
                n1358 = property class="Arr (strict)"(reference=w1807) -> ("Value"=w1803:i32[])  [unwired: 1 in, 2 out]
                n1359 = Build Array(w1809, w1808) -> (w1819:dbl[])
                n1360 = call "camToStage_abs_3d.vi"("transform cluster + actuator"=w1820, "abs pixel location"=w1819) -> ("pipette location (steps)"=w1805:dbl[])  [unwired: 9 in]
                n1361 = Index Array(array=w1803) -> (element #1=w1802:i32, element #2=w1798:i32, element #3=w1804:i32)  [unwired: 3 in]
                n1362 = Unbundle By Name(w1820) -> ("s"=w1824:refnum<vi>)
                n1363 = Index Array(array=w1805) -> (element #1=w1801:dbl, element #2=w1797:dbl)  [unwired: 3 in, 1 out]
                n1364 = Subtract(x=w1802, y=w1801) -> (x-y=w1800:dbl)
                n1365 = Subtract(x=w1798, y=w1797) -> (x-y=w1799:dbl)
                n1366 = property class="Clust (strict)"(reference=w1824) -> ("Value"=w1823:T25)  [unwired: 1 in, 2 out]
                n1367 = Build Array(w1800, w1799, w1804) -> (w1796:dbl[])
                n1368 = Unbundle By Name(w1823) -> ("actuator"=w1822:T26)
                n1369 = call "moveTo_abs_XYZ.vi"("blocking?"=TRUE, "XYZ location (steps)"=w1796, "Actuator cluster in"=w1822) -> ()  [unwired: 7 in, 2 out]
              }
            }
          }
          frame "Pipette template" {
            w1827 = 0 items=["All", "Low Discrepancy Sampling", "Grayscale Value Pyramid", "Gradients Pyramid"] ("Algorithm")
            # "corrMask"
            n1370 = case shown="\"manipulator 1\", Default" w1846 {
              tunnel: [w1886 w1893] -> w1862
              tunnel: ["pipette 1 cell tracker rectangle" "pipette 2 cell tracker rectangle"] -> w1841
              tunnel: [w1883 w1888] -> w1856
              tunnel: [w1881 w1889] -> w1855
              tunnel: [w1882 w1892] -> w1854
              tunnel: [w1884 w1891] -> w1830
              tunnel: w1853 -> [w1884 _]
              tunnel: w1852 -> [w1882 _]
              tunnel: w1851 -> [_ w1892]
              tunnel: w1850 -> [w1883 _]
              tunnel: w1849 -> [w1881 _]
              tunnel: w1848 -> [_ w1889]
              tunnel: w1847 -> [_ w1888]
              tunnel: w1844 -> [_ w1891]
              tunnel: w1840 -> [w1880 _]
              tunnel: w1839 -> [_ w1887]
              tunnel: [w1880 w1887] -> w1838
              frame "manipulator 1", Default {
                n1371 = local read "manip 1 position"() -> (w1886:T23)
                n1372 = local write "pipette 1 mask"(w1884) -> ()
              }
              frame "manipulator 2" {
                n1373 = local read "manip 2 position"() -> (w1893:T23)
                n1374 = local write "pipette mask 2"(w1891) -> ()
              }
            }
            n1375 = Unbundle By Name(w1863) -> ("X"=w1867:i32, "Y"=w1866:i32)
            n1376 = call "IMAQ Clear Overlay"("Image"=w1826) -> ("error out"=w1868:errorcluster, "Image Out"=w1869:T10)  [unwired: 9 in]
            n1377 = Build Array(w1867, w1866) -> (w1865:i32[])
            n1378 = call "makeOuterMaskBox.vi"("manip 1 position"=w1862, "user selected pipette tip (x,y)"=w1865) -> ("bounding rectangle"=w1864:i32[])  [unwired: 8 in, 1 out]
            n1379 = call "IMAQ Extract 2"("Optional Rectangle"=w1864, "error in (no error)"=w1868, "Image Dst"=w1854, "Image Src"=w1869) -> ("error out"=w1829:errorcluster, "Image Dst Out"=w1831:T10)  [unwired: 6 in]
            n1380 = call "IMAQ Learn Pattern 5"("Image"=w1831, "Algorithm"=w1827, "Mask"=w1830, "error in (no error)"=w1829) -> ("Template Image Out"=w1832:T10, "error out"=w1828:errorcluster)  [unwired: 9 in, 1 out]
            n1381 = call-poly "IMAQ Write File 2"("error in (no error)"=w1828, "File Path"=w1856, "Image"=w1832) -> ("error out"=w1859:errorcluster)  [unwired: 7 in, 1 out]
            n1382 = call "IMAQ Extract 2"("Optional Rectangle"=w1841, "error in (no error)"=w1859, "Image Dst"=w1855, "Image Src"=w1832) -> ("error out"=w1843:errorcluster, "Image Dst Out"=w1858:T10)  [unwired: 6 in]
            n1383 = call "IMAQ Extract 2"("Optional Rectangle"=w1841, "error in (no error)"=w1843, "Image Dst"=w1838, "Image Src"=w1830) -> ("error out"=w1842:errorcluster, "Image Dst Out"=w1837:T10)  [unwired: 6 in]
            "pipette corrMask" <- w1837
            n1384 = local read "cell tracker"() -> (w1833:bool)
            n1385 = call <vilib>:"Simple Error Handler.vi"("error in (no error)"=w1842) -> ("error out"=w1870:errorcluster)  [unwired: 4 in, 4 out]
            n1386 = call <vilib>:"Clear Errors.vi"("error in (no error)"=w1870) -> ("error out"=w1860:errorcluster)  [unwired: 5 in, 1 out]
            n1387 = call "IMAQ ImageToArray"("error in (no error)"=w1860, "Image"=w1858) -> ("error out"=w1835:errorcluster, "Image Pixels (U8)"=w1861:u8[][])  [unwired: 2 in, 3 out]
            n1388 = call "IMAQ ImageToArray"("error in (no error)"=w1835, "Image"=w1837) -> ("error out"=w1834:errorcluster, "Image Pixels (U8)"=w1836:u8[][])  [unwired: 2 in, 3 out]
            n1389 = case shown="True" w1833 {
              tunnel: w1861 -> [_ w1875]
              tunnel: [w1871 w1874] -> w1857
              tunnel: w1836 -> [_ w1873]
              tunnel: w1834 -> [w1871 w1872]
              frame False {
              }
              frame True {
                n1390 = script code="clearvars -except pipette_image pipette_corrMask;\n\n[Pipette_seg, Pipette_tip] = userdrawPipetteSegmentation(pipette_image);"("??"=w1872, "pipette_image"=w1875, "pipette_corrMask"=w1873) -> ("??"=w1874:errorcluster)
              }
            }
            "tip select error" <- w1857
            n1391 = case shown="\"manipulator 1\", Default" w1845 {
              tunnel: w1832 -> [w1877 w1878]
              tunnel: w1858 -> [w1876 w1879]
              frame "manipulator 1", Default {
                n1392 = local write "pipette 1 template"(w1877) -> ()
                "pipette 1 mask for cell tracker" <- w1876
              }
              frame "manipulator 2" {
                n1393 = local write "pipette 2 template"(w1878) -> ()
                "pipette 2 mask for cell tracker" <- w1879
              }
            }
          }
          frame "none" {
          }
        }
      }
      event "cell autofocus": Value Change {
        n1394 = event-data() -> ("NewVal"=w1900:bool)  [unwired: 1 in, 5 out]
        n1395 = Unbundle By Name(w1895) -> ("s"=w1899:refnum<vi>)
        n1396 = property class="Clust (strict)"(reference=w1899) -> ("Value"=w1898:T25)  [unwired: 1 in, 2 out]
        n1397 = Unbundle By Name(w1898) -> ("actuator"=w1897:T26)
        n1398 = case shown="True" w1900 {
          tunnel: w1896 -> [_ w1909]
          tunnel: w1897 -> [_ w1908]
          tunnel: w1895 -> [_ w1901]
          frame False {
          }
          frame True {
            n1399 = local read "cell match score"() -> (w1906:sgl)
            n1400 = local read "cell images"() -> (w1903:T10[])
            n1401 = local read "index"() -> (w1907:i32)
            n1402 = call "stageFindCell_v5.vi"("stage in"=w1908, "slice image"=w1909, "cell index"=w1907, "transform cluster + actuator"=w1901, "cell match score"=w1906, "cell images"=w1903) -> ("cell found"=→"cell found?":bool, "screen cell location (px)"=w1904:i32[], "Score"=→"cell score":sgl)  [unwired: 4 in, 3 out]
            n1403 = local write "screen tip location (px)"(w1904) -> ()
          }
        }
      }
      event "MATLAB clearvars": Value Change {
        n1404 = event-data() -> ("NewVal"=w1911:bool)  [unwired: 1 in, 5 out]
        n1405 = case shown="True" w1911 {
          frame False {
          }
          frame True {
            n1406 = script code="clearvars"() -> ()  [unwired: 1 in, 1 out]
          }
        }
      }
      event "go to cell index": Value Change {
        n1407 = event-data() -> ("NewVal"=w1916:bool)  [unwired: 1 in, 5 out]
        n1408 = case shown="True" w1916 {
          tunnel: w1913 -> [_ w1926]
          tunnel: w1915 -> [_ w1920]
          tunnel: w1914 -> [_ w1919]
          frame False {
          }
          frame True {
            n1409 = local read "current cell locations (px)"() -> (w1927:dbl[][])
            n1410 = call "get_screenCenter.vi"("use demo values?"=FALSE, "image"=w1926) -> ("screen center (px)"=w1922:i32[])  [unwired: 9 in]
            n1411 = Transpose 2D Array(2D array=w1927) -> (transposed array=w1929:dbl[][])
            n1412 = Index Array(array=w1929, index (row)="index") -> (element=w1923:dbl[])  [unwired: 1 in]
            n1413 = call "stageToCam.vi"("center location"=w1922, "transform cluster + actuator"=w1919, "current positions"=w1920, "cam location (px)"=w1923) -> ("stage location (steps)"=w1921:dbl[])  [unwired: 6 in, 1 out]
            n1414 = case shown="False" "backlash?" {
              tunnel: w1923 -> [_ w1940]
              tunnel: w1922 -> [_ w1937]
              tunnel: w1920 -> [_ w1935]
              tunnel: w1919 -> [_ w1934]
              tunnel: [errorcluster {"status"=FALSE, "code"=0, "source"=""} ("error out") w1931] -> w1917
              frame False {
              }
              frame True {
                n1415 = Subtract(x=w1940, y=dbl[] [100.0, 100.0, 0.0]) -> (x-y=w1938:dbl[])
                n1416 = call "stageToCam.vi"("center location"=w1937, "transform cluster + actuator"=w1934, "current positions"=w1935, "cam location (px)"=w1938) -> ("stage location (steps)"=w1936:dbl[])  [unwired: 6 in, 1 out]
                n1417 = call "move stage abs.vi"("blocking?"=TRUE, "transform cluster + actuator"=w1934, "positions"=w1935, "location (steps)"=w1936) -> ("error out"=w1932:errorcluster)  [unwired: 7 in]
                n1418 = call "Time Delay24"("error in (no error)"=w1932, "Delay Time (s)"=1.0) -> ("error out"=w1931:errorcluster)  [unwired: 9 in]
              }
            }
            n1419 = call "move stage abs.vi"("blocking?"=TRUE, "error in (no error)"=w1917, "transform cluster + actuator"=w1919, "positions"=w1920, "location (steps)"=w1921) -> ()  [unwired: 6 in, 1 out]
          }
        }
      }
      event "User OK": Value Change {
        n1420 = event-data() -> ()  [unwired: 1 in, 6 out]
        n1421 = disable-structure shown="Disabled" {
          frame Disabled {
            n1422 = control-ref of="Pane"() -> (w1943:refnum<vi>)
            n1423 = property class="Pane"(reference=w1943) -> ("Controls[]"=w1942:refnum<vi>[])  [unwired: 1 in, 2 out]
            n1424 = local write "allMainVIcontrols"(w1942) -> ()
          }
          frame Enabled {
          }
        }
      }
      event "zero stage measurement": Value Change {
        n1425 = event-data() -> ("NewVal"=w1945:bool)  [unwired: 1 in, 5 out]
        n1426 = case shown="True" w1945 {
          frame False {
          }
          frame True {
            n1427 = local read "current stage pos (steps)"() -> (w1946:i32[])
            n1428 = local write "measured stage zero (steps)"(w1946) -> ()
          }
        }
      }
      event "zero manip measurement": Value Change {
        n1429 = event-data() -> ("NewVal"=w1948:bool)  [unwired: 1 in, 5 out]
        n1430 = case shown="True" w1948 {
          frame False {
          }
          frame True {
            n1431 = local read "current manip 1 pos (steps)"() -> (w1949:i32[])
            n1432 = local write "measured manip 1 zero (steps)"(w1949) -> ()
          }
        }
      }
      event "test multiclamp": Value Change {
        n1433 = event-data() -> ("NewVal"=w1952:bool)  [unwired: 1 in, 5 out]
        n1434 = case shown="True" w1952 {
          tunnel: w1951 -> [_ w1957]
          frame False {
          }
          frame True {
            w1953 = u32 0 ("ModeConstant")
            n1435 = dll-call lib="C:/multiBot/patcherBot/AxMultiClampMsg.dll" fn="MCCMSG_SetMode"("handle"=w1957, "ModeConstant"=w1953, "error"=w1953) -> ("error"=w1956:i32)  [unwired: 6 in, 2 out]
            n1436 = Not Equal To 0?(x=w1956) -> (x != 0?=w1954:bool)
            n1437 = Not(x=w1954) -> (.not. x?=w1955:bool)
            n1438 = call "Display Message to User"("Enable"=w1954) -> ()  [unwired: 9 in, 2 out]
            n1439 = local write "multiclamp on"(w1955) -> ()
          }
        }
      }
      event "empty list", "delete location": Value Change {
        n1440 = event-data() -> ("OldVal"=w1961:bool, "NewVal"=w1960:bool)  [unwired: 1 in, 4 out]
        n1441 = Not And(1:w1960, 2:w1961) -> (0:w1962:bool)
        n1442 = Select(t=w1960, s=w1962, f=w1961) -> (s? t:f=w1959:bool)
        n1443 = case shown="True" w1959 {
          tunnel: [w1966 w1974] -> w1964
          tunnel: [w1965 w1970] -> w1963
          frame False {
            n1444 = local read "cells (image px)"() -> (w1966:dbl[][])
            n1445 = local read "cell images"() -> (w1965:T10[])
          }
          frame True {
            n1446 = local read "cells (image px)"() -> (w1973:dbl[][])
            n1447 = local read "cell images"() -> (w1971:T10[])
            n1448 = local read "index"() -> (w1972:i32)
            n1449 = local read "unpatched+reserved"() -> (w1969:i32[])
            n1450 = local read "empty list"() -> (w1967:bool)
            n1451 = case shown="False" w1967 {
              tunnel: [w1980 dbl[][] [] ("cell positions (stage steps)")] -> w1974
              tunnel: w1973 -> [w1981 _]
              tunnel: w1972 -> [w1976 _]
              tunnel: w1971 -> [w1979 _]
              tunnel: [w1978 T10[] [] ("cell images")] -> w1970
              tunnel: w1969 -> [w1977 _]
              tunnel: [w1975 i32[] [] ("unpatched+reserved")] -> w1968
              frame False {
                # "delete cell"
                n1452 = Delete From Array(array=w1977, index=w1976) -> (array with subset deleted=w1975:i32[])  [unwired: 1 in, 1 out]
                n1453 = Delete From Array(array=w1981, index (col)=w1976) -> (array with subset deleted=w1980:dbl[][])  [unwired: 2 in, 1 out]
                n1454 = Delete From Array(array=w1979, index=w1976) -> (array with subset deleted=w1978:T10[])  [unwired: 1 in, 1 out]
              }
              frame True {
                # "empty array"
              }
            }
            n1455 = local write "unpatched+reserved"(w1968) -> ()
          }
        }
        n1456 = local write "cells (image px)"(w1964) -> ()
        n1457 = local write "cell images"(w1963) -> ()
      }
      event "location above baths", "wash bath location", "cleaning bath location": Value Change {
        n1458 = event-data() -> ("NewVal"=w1987:bool)  [unwired: 1 in, 5 out]
        n1459 = case shown="True" w1987 {
          tunnel: w1986 -> [_ w1991]
          frame False {
          }
          frame True {
            n1460 = disable-structure shown="Disabled" {
              disable-tunnel: [w1997 _] -> _
              frame Disabled {
                n1461 = local read "cleaning tab"() -> (w1997:enum32{"manip 1", "manip 2"})
              }
              frame Enabled {
              }
            }
            n1462 = local read "Calibrate:"() -> (w1989:T8)
            n1463 = case shown="\"manipulator 2\"" w1989 {
              tunnel: [w1998 w2001] -> w1992
              tunnel: w1991 -> [w1999 w2000]
              frame "manipulator 1", Default {
                n1464 = Unbundle By Name(w1999) -> ("manip 1"=w1998:refnum<vi>)
              }
              frame "manipulator 2" {
                n1465 = Unbundle By Name(w2000) -> ("manip 2"=w2001:refnum<vi>)
              }
            }
            n1466 = property class="Clust (strict)"(reference=w1992) -> ("Value"=w1990:T25)  [unwired: 1 in, 2 out]
            n1467 = Unbundle By Name(w1990) -> ("actuator"=w1988:T26)